vi "UHR-Fleezers Control (host) - Avogadro v2.vi"() -> ()   [LabVIEW 2014] (continued)
                                n2721 = local read "Confocal Y 1 (V)"() -> (w4187:dbl)
                                n2722 = property on="AO2" class="Slide (strict)"("Val(Sgnl)"=w4186) -> ()  [unwired: 2 in, 2 out]
                                n2723 = property on="AO1" class="Slide (strict)"("Val(Sgnl)"=w4187) -> ()  [unwired: 2 in, 2 out]
                                }
                                }
                                }
                                }
                                }
                                }
                                }
                                }
                                }
                                frame "Image" {
                                n2724 = property on="Confocal Image" class="Bool (strict)"("Val(Sgnl)"=TRUE ("Value (Signaling)")) -> ()  [unwired: 2 in, 2 out]
                                }
                              }
                              n2725 = local write "Fl. High"(FALSE ("Fl. High")) -> ()
                              n2726 = local read "Time (s)"() -> (w4123:dbl)
                            }
                            frame #1 {
                              n2727 = case shown="True" "Auto F Reset" {
                                tunnel: w4195 -> [_ w4200]
                                tunnel: w4194 -> [_ w4199]
                                tunnel: w4193 -> [_ w4198]
                                tunnel: w4192 -> [_ w4197]
                                frame False {
                                }
                                frame True {
                                n2728 = node-c288() -> (w4202:T42)  [unwired: 4 in]
                                n2729 = timed-loop {
                                timing: w4202 -> [_]
                                timing-out: [_] -> w4201
                                tunnel: w4200 -> [w4207]
                                tunnel: w4199 -> [w4206]
                                tunnel: w4198 -> [w4205]
                                tunnel: w4197 -> [w4204]
                                stop <- w4203 stop-if-true
                                n2730 = node-c288() -> ()  [unwired: 1 in, 1 out]
                                n2731 = local read "Fl. Delta Thresh. (kHz)"() -> (w4216:dbl)
                                n2732 = local read "APD to Watch"() -> (w4217:bool)
                                n2733 = local read "Delta Fl. 1"() -> (w4218:dbl)
                                n2734 = local read "Delta Fl. 2"() -> (w4219:dbl)
                                n2735 = local read "Fl. Triggered..."() -> (w4210:bool)
                                n2736 = local read "Stop All"() -> (w4211:bool)
                                n2737 = local read "Reset Force"() -> (w4209:bool)
                                n2738 = Multiply(x=w4216, y=1000.0) -> (x*y=w4214:dbl)
                                n2739 = Select(t=w4218, s=w4217, f=w4219) -> (s? t:f=w4213:dbl)
                                n2740 = Not(x=w4210) -> (.not. x?=w4208:bool)
                                n2741 = Greater?(x=w4213, y=w4214) -> (0:w4212:bool)
                                n2742 = Compound Arithmetic op=OR(w4212, w4211, w4208, w4209) -> (w4203:bool)
                                n2743 = case shown="True" w4203 {
                                tunnel: w4207 -> [_ w4223]
                                tunnel: w4206 -> [_ w4227]
                                tunnel: w4205 -> [_ w4226]
                                tunnel: w4204 -> [_ w4225]
                                frame False {
                                }
                                frame True {
                                n2744 = case shown="\"Yank\"" w4227 {
                                tunnel: w4226 -> [_ w4237]
                                tunnel: w4225 -> [_ w4235]
                                frame "Image", Default {
                                }
                                frame "Yank" {
                                n2745 = flat-sequence {
                                tunnel: [w4240] -> w4238
                                tunnel: w4237 -> [w4240]
                                tunnel: [w4239] -> w4236
                                tunnel: w4235 -> [w4239]
                                tunnel: w4238 -> [w4246]
                                tunnel: w4236 -> [w4244]
                                frame #0 {
                                n2746 = local read "Yank Delay (s)"() -> (w4243:dbl)
                                n2747 = Multiply(x=w4243, y=1000.0) -> (x*y=w4241:dbl)
                                n2748 = Wait (ms)(milliseconds to wait=w4241) -> ()  [unwired: 1 out]
                                }
                                frame #1 {
                                n2749 = local read "Yank to which?"() -> (w4245:bool)
                                n2750 = case shown="False" w4245 {
                                tunnel: w4246 -> [_ w4274]
                                tunnel: w4244 -> [w4247 _]
                                frame False {
                                n2751 = flat-sequence {
                                tunnel: w4247 -> [w4248]
                                frame #0 {
                                n2752 = property on="Trap Pos FB SP" class="DigNum (strict)"("Val(Sgnl)"=w4248) -> ()  [unwired: 2 in, 2 out]
                                }
                                frame #1 {
                                n2753 = Wait (ms)(milliseconds to wait=u32 700) -> ()  [unwired: 1 out]
                                }
                                frame #2 {
                                n2754 = local read "Action (%)"() -> (w4253:dbl)
                                n2755 = Absolute Value(x=w4253) -> (abs(x)=w4252:dbl)
                                n2756 = Greater?(x=w4252, y=70.0) -> (0:w4250:bool)
                                n2757 = property on="Remove Action Offset" class="Bool (strict)"("Val(Sgnl)"=w4250) -> ()  [unwired: 2 in, 2 out]
                                }
                                frame #3 {
                                n2758 = for {
                                N: 4 -> [_]
                                n2759 = flat-sequence {
                                frame #0 {
                                n2760 = Wait (ms)(milliseconds to wait=u32 500) -> ()  [unwired: 1 out]
                                }
                                frame #1 {
                                n2761 = local read "Action (%)"() -> (w4259:dbl)
                                n2762 = Absolute Value(x=w4259) -> (abs(x)=w4258:dbl)
                                n2763 = Greater?(x=w4258, y=70.0) -> (0:w4256:bool)
                                n2764 = property on="Remove Action Offset" class="Bool (strict)"("Val(Sgnl)"=w4256) -> ()  [unwired: 2 in, 2 out]
                                }
                                }
                                }
                                }
                                frame #4 {
                                n2765 = Wait (ms)(milliseconds to wait=u32 500) -> ()  [unwired: 1 out]
                                }
                                frame #5 {
                                n2766 = local read "Shift confocal"() -> (w4264:bool)
                                n2767 = local read "Mean"() -> (w4267:dbl)
                                n2768 = Greater?(x=w4267, y=11.0) -> (0:w4263:bool)
                                n2769 = Not(x=w4263) -> (.not. x?=w4262:bool)
                                n2770 = And(x=w4263, y=w4264) -> (x .and. y?=w4265:bool)
                                n2771 = And(x=w4262, y=w4264) -> (x .and. y?=w4261:bool)
                                n2772 = case shown="True" w4265 {
                                frame False {
                                }
                                frame True {
                                n2773 = local read "Confocal X 2 (V)"() -> (w4270:dbl)
                                n2774 = local read "Confocal Y 2 (V)"() -> (w4271:dbl)
                                n2775 = property on="AO2" class="Slide (strict)"("Val(Sgnl)"=w4270) -> ()  [unwired: 2 in, 2 out]
                                n2776 = property on="AO1" class="Slide (strict)"("Val(Sgnl)"=w4271) -> ()  [unwired: 2 in, 2 out]
                                }
                                }
                                n2777 = case shown="True" w4261 {
                                frame False {
                                }
                                frame True {
                                n2778 = local read "Confocal Y 1 (V)"() -> (w4269:dbl)
                                n2779 = local read "Confocal X 1 (V)"() -> (w4268:dbl)
                                n2780 = property on="AO1" class="Slide (strict)"("Val(Sgnl)"=w4269) -> ()  [unwired: 2 in, 2 out]
                                n2781 = property on="AO2" class="Slide (strict)"("Val(Sgnl)"=w4268) -> ()  [unwired: 2 in, 2 out]
                                }
                                }
                                }
                                frame #6 {
                                n2782 = Wait (ms)(milliseconds to wait=u32 1500) -> ()  [unwired: 1 out]
                                }
                                frame #7 {
                                n2783 = property on="Rem fb disp offset" class="Bool (strict)"("Val(Sgnl)"=TRUE ("Value (Signaling)")) -> ()  [unwired: 2 in, 2 out]
                                }
                                }
                                }
                                frame True {
                                n2784 = flat-sequence {
                                tunnel: w4274 -> [w4275]
                                frame #0 {
                                n2785 = property on="Trap Delta (MHz)" class="DigNum (strict)"("Val(Sgnl)"=w4275) -> ()  [unwired: 2 in, 2 out]
                                }
                                frame #1 {
                                n2786 = Wait (ms)(milliseconds to wait=u32 500) -> ()  [unwired: 1 out]
                                }
                                frame #2 {
                                n2787 = local read "Shift confocal"() -> (w4281:bool)
                                n2788 = local read "Mean"() -> (w4282:dbl)
                                n2789 = Greater?(x=w4282, y=11.0) -> (0:w4280:bool)
                                n2790 = And(x=w4280, y=w4281) -> (x .and. y?=w4278:bool)
                                n2791 = Not(x=w4280) -> (.not. x?=w4279:bool)
                                n2792 = And(x=w4279, y=w4281) -> (x .and. y?=w4277:bool)
                                n2793 = case shown="True" w4278 {
                                frame False {
                                }
                                frame True {
                                n2794 = local read "Confocal Y 2 (V)"() -> (w4287:dbl)
                                n2795 = local read "Confocal X 2 (V)"() -> (w4286:dbl)
                                n2796 = property on="AO1" class="Slide (strict)"("Val(Sgnl)"=w4287) -> ()  [unwired: 2 in, 2 out]
                                n2797 = property on="AO2" class="Slide (strict)"("Val(Sgnl)"=w4286) -> ()  [unwired: 2 in, 2 out]
                                }
                                }
                                n2798 = case shown="True" w4277 {
                                frame False {
                                }
                                frame True {
                                n2799 = local read "Confocal Y 1 (V)"() -> (w4285:dbl)
                                n2800 = local read "Confocal X 1 (V)"() -> (w4284:dbl)
                                n2801 = property on="AO2" class="Slide (strict)"("Val(Sgnl)"=w4284) -> ()  [unwired: 2 in, 2 out]
                                n2802 = property on="AO1" class="Slide (strict)"("Val(Sgnl)"=w4285) -> ()  [unwired: 2 in, 2 out]
                                }
                                }
                                }
                                }
                                }
                                }
                                }
                                }
                                }
                                }
                                n2803 = local read "Time (s)"() -> (w4222:dbl)
                                n2804 = Subtract(x=w4223, y=w4222) -> (x-y=w4234:dbl)
                                n2805 = Number To Decimal String(number=w4234, width (-)=i16 0) -> (decimal integer string=w4232:string)
                                n2806 = Concatenate Strings(w4232, " s fluorescence event") -> (w4229:string)
                                n2807 = local read "Messages"() -> (w4230:string)
                                n2808 = local write "Duration (s)"(w4234) -> ()
                                n2809 = call "Update messages.vi"("Message to add"=w4229, "Old message string"=w4230) -> ("New message string"=w4228:string)
                                n2810 = local write "Messages"(w4228) -> ()
                                n2811 = call <vilib>:"Beep.vi"() -> ()  [unwired: 12 in]
                                n2812 = local write "Reset Force"(FALSE ("Force Reset")) -> ()
                                n2813 = local write "Fl. High"(TRUE ("Fl. High")) -> ()
                                n2814 = local write "Waiting"(TRUE ("Waiting")) -> ()
                                }
                                }
                                n2815 = node-c288() -> ()  [unwired: 1 in, 1 out]
                                }
                                n2816 = node-c288(w4201) -> ()  [unwired: 1 out]
                                }
                              }
                            }
                          }
                          n2817 = local read "Trap Delta (MHz)"() -> (w4113:dbl)
                          n2818 = local read "Trap Pos FB SP"() -> (w4111:fxp<+/-,16,1>)
                        }
                      }
                    }
                    frame True {
                      n2819 = flat-sequence {
                        tunnel: w4298 -> [w4308]
                        tunnel: [w4308] -> w4302
                        tunnel: w4301 -> [w4307]
                        tunnel: [w4307] -> w4300
                        tunnel: [w4306] -> w4299
                        tunnel: w4297 -> [w4305]
                        tunnel: [w4304] -> w4296
                        tunnel: w4293 -> [w4303]
                        tunnel: [w4303] -> w4292
                        tunnel: w4302 -> [w4378]
                        tunnel: w4300 -> [w4377]
                        tunnel: w4299 -> [w4376]
                        tunnel: w4296 -> [w4375]
                        tunnel: w4292 -> [w4374]
                        tunnel: [w4375] -> w4295
                        frame #0 {
                          n2820 = call <vilib>:"Beep.vi"() -> ()  [unwired: 3 in, 9 out]
                          n2821 = local write "Waiting"(FALSE ("Waiting")) -> ()
                          n2822 = Increment(x=w4305) -> (x+1=w4304:u8)
                          n2823 = case shown="\"Image\"" w4307 {
                            tunnel: w4304 -> [_ _ w4314]
                            frame "Image" {
                              n2824 = property on="Confocal Image" class="Bool (strict)"("Val(Sgnl)"=TRUE ("Value (Signaling)")) -> ()  [unwired: 2 in, 2 out]
                            }
                            frame "Alarm", Default {
                            }
                            frame "Yank" {
                              n2825 = flat-sequence {
                                tunnel: w4314 -> [w4317]
                                tunnel: [w4316] -> w4313
                                tunnel: ["N Array El"] -> w4312
                                tunnel: w4313 -> [w4331]
                                tunnel: w4312 -> [w4327]
                                frame #0 {
                                n2826 = Multiply(x="Yank Delay (s)", y=1000.0) -> (x*y=w4320:dbl)
                                n2827 = Quotient & Remainder(x=w4317, y="N Array El") -> (x-y*floor(x/y)=w4316:u8)  [unwired: 1 out]
                                n2828 = Wait (ms)(milliseconds to wait=w4320) -> ()  [unwired: 1 out]
                                }
                                frame #1 {
                                n2829 = Random Number (0-1)() -> (number: 0 to 1=w4328:dbl)
                                n2830 = Multiply(x=w4327, y=w4328) -> (x*y=w4326:dbl)
                                n2831 = Round Toward -Infinity(1:w4326) -> (0:w4325:dbl)
                                n2832 = Select(t=w4325, s="Random Choice", f=w4331) -> (s? t:f=w4329:dbl)
                                n2833 = Select(t="Yank to Trap Delta (MHz)", s="Yank to which?", f="Yank to SP") -> (s? t:f=w4322:dbl[])
                                n2834 = Index Array(array=w4322, index=w4329) -> (element=w4332:dbl)
                                n2835 = case shown="False" "Yank to which?" {
                                tunnel: w4332 -> [w4333 w4359]
                                frame False {
                                n2836 = flat-sequence {
                                tunnel: w4333 -> [w4334]
                                frame #0 {
                                n2837 = property on="Trap Pos FB SP" class="DigNum (strict)"("Val(Sgnl)"=w4334) -> ()  [unwired: 2 in, 2 out]
                                }
                                frame #1 {
                                n2838 = Wait (ms)(milliseconds to wait=u32 700) -> ()  [unwired: 1 out]
                                }
                                frame #2 {
                                n2839 = local read "Action (%)"() -> (w4339:dbl)
                                n2840 = Absolute Value(x=w4339) -> (abs(x)=w4338:dbl)
                                n2841 = Greater?(x=w4338, y=70.0) -> (0:w4336:bool)
                                n2842 = property on="Remove Action Offset" class="Bool (strict)"("Val(Sgnl)"=w4336) -> ()  [unwired: 2 in, 2 out]
                                }
                                frame #3 {
                                n2843 = for {
                                N: 4 -> [_]
                                n2844 = flat-sequence {
                                frame #0 {
                                n2845 = Wait (ms)(milliseconds to wait=u32 500) -> ()  [unwired: 1 out]
                                }
                                frame #1 {
                                n2846 = local read "Action (%)"() -> (w4345:dbl)
                                n2847 = Absolute Value(x=w4345) -> (abs(x)=w4344:dbl)
                                n2848 = Greater?(x=w4344, y=70.0) -> (0:w4342:bool)
                                n2849 = property on="Remove Action Offset" class="Bool (strict)"("Val(Sgnl)"=w4342) -> ()  [unwired: 2 in, 2 out]
                                }
                                }
                                }
                                }
                                frame #4 {
                                n2850 = local read "Shift confocal"() -> (w4349:bool)
                                n2851 = local read "Mean"() -> (w4352:dbl)
                                n2852 = Greater?(x=w4352, y=11.0) -> (0:w4348:bool)
                                n2853 = Not(x=w4348) -> (.not. x?=w4347:bool)
                                n2854 = And(x=w4347, y=w4349) -> (x .and. y?=w4346:bool)
                                n2855 = And(x=w4348, y=w4349) -> (x .and. y?=w4350:bool)
                                n2856 = case shown="True" w4350 {
                                frame False {
                                }
                                frame True {
                                n2857 = local read "Confocal X 2 (V)"() -> (w4355:dbl)
                                n2858 = local read "Confocal Y 2 (V)"() -> (w4356:dbl)
                                n2859 = property on="AO2" class="Slide (strict)"("Val(Sgnl)"=w4355) -> ()  [unwired: 2 in, 2 out]
                                n2860 = property on="AO1" class="Slide (strict)"("Val(Sgnl)"=w4356) -> ()  [unwired: 2 in, 2 out]
                                }
                                }
                                n2861 = case shown="True" w4346 {
                                frame False {
                                }
                                frame True {
                                n2862 = local read "Confocal X 1 (V)"() -> (w4353:dbl)
                                n2863 = local read "Confocal Y 1 (V)"() -> (w4354:dbl)
                                n2864 = property on="AO1" class="Slide (strict)"("Val(Sgnl)"=w4354) -> ()  [unwired: 2 in, 2 out]
                                n2865 = property on="AO2" class="Slide (strict)"("Val(Sgnl)"=w4353) -> ()  [unwired: 2 in, 2 out]
                                }
                                }
                                }
                                frame #5 {
                                n2866 = Wait (ms)(milliseconds to wait=u32 1500) -> ()  [unwired: 1 out]
                                }
                                frame #6 {
                                n2867 = property on="Rem fb disp offset" class="Bool (strict)"("Val(Sgnl)"=TRUE ("Value (Signaling)")) -> ()  [unwired: 2 in, 2 out]
                                }
                                }
                                }
                                frame True {
                                n2868 = flat-sequence {
                                tunnel: w4359 -> [w4360]
                                frame #0 {
                                n2869 = property on="Trap Delta (MHz)" class="DigNum (strict)"("Val(Sgnl)"=w4360) -> ()  [unwired: 2 in, 2 out]
                                }
                                frame #1 {
                                n2870 = Wait (ms)(milliseconds to wait=u32 500) -> ()  [unwired: 1 out]
                                }
                                frame #2 {
                                n2871 = local read "Shift confocal"() -> (w4364:bool)
                                n2872 = local read "Mean"() -> (w4362:dbl)
                                n2873 = Greater?(x=w4362, y=11.0) -> (0:w4365:bool)
                                n2874 = Not(x=w4365) -> (.not. x?=w4366:bool)
                                n2875 = And(x=w4366, y=w4364) -> (x .and. y?=w4368:bool)
                                n2876 = And(x=w4365, y=w4364) -> (x .and. y?=w4367:bool)
                                n2877 = case shown="True" w4367 {
                                frame False {
                                }
                                frame True {
                                n2878 = local read "Confocal Y 2 (V)"() -> (w4372:dbl)
                                n2879 = local read "Confocal X 2 (V)"() -> (w4371:dbl)
                                n2880 = property on="AO1" class="Slide (strict)"("Val(Sgnl)"=w4372) -> ()  [unwired: 2 in, 2 out]
                                n2881 = property on="AO2" class="Slide (strict)"("Val(Sgnl)"=w4371) -> ()  [unwired: 2 in, 2 out]
                                }
                                }
                                n2882 = case shown="True" w4368 {
                                frame False {
                                }
                                frame True {
                                n2883 = local read "Confocal X 1 (V)"() -> (w4369:dbl)
                                n2884 = local read "Confocal Y 1 (V)"() -> (w4370:dbl)
                                n2885 = property on="AO2" class="Slide (strict)"("Val(Sgnl)"=w4369) -> ()  [unwired: 2 in, 2 out]
                                n2886 = property on="AO1" class="Slide (strict)"("Val(Sgnl)"=w4370) -> ()  [unwired: 2 in, 2 out]
                                }
                                }
                                }
                                }
                                }
                                }
                                }
                              }
                            }
                          }
                          n2887 = local read "Time (s)"() -> (w4306:dbl)
                          "Fl. High" <- TRUE ("Yanking")
                        }
                        frame #1 {
                          n2888 = local read "Auto F Reset"() -> (w4373:bool)
                          n2889 = case shown="True" w4373 {
                            tunnel: w4378 -> [_ w4382]
                            tunnel: w4377 -> [_ w4381]
                            tunnel: w4376 -> [_ w4380]
                            tunnel: w4374 -> [_ w4379]
                            frame False {
                            }
                            frame True {
                              n2890 = node-c288() -> (w4384:T42)  [unwired: 4 out]
                              n2891 = timed-loop {
                                timing: w4384 -> [_]
                                timing-out: [_] -> w4383
                                tunnel: w4382 -> [w4402]
                                tunnel: w4381 -> [w4401]
                                tunnel: w4380 -> [w4400]
                                tunnel: w4379 -> [w4399]
                                stop <- w4385 stop-if-true
                                n2892 = node-c288() -> ()  [unwired: 2 out]
                                n2893 = local read "Fl. Delta Thresh. (kHz)"() -> (w4393:dbl)
                                n2894 = local read "Fl. Triggered..."() -> (w4398:bool)
                                n2895 = local read "Delta Fl. 1"() -> (w4389:dbl)
                                n2896 = local read "Delta Fl. 2"() -> (w4387:dbl)
                                n2897 = local read "Stop All"() -> (w4396:bool)
                                n2898 = local read "APD to Watch"() -> (w4388:bool)
                                n2899 = Select(t=w4389, s=w4388, f=w4387) -> (s? t:f=w4386:dbl)
                                n2900 = Not(x=w4398) -> (.not. x?=w4397:bool)
                                n2901 = Multiply(x=w4393, y=1000.0) -> (x*y=w4392:dbl)
                                n2902 = Negate(x=w4392) -> (-x=w4391:dbl)
                                n2903 = Less?(x=w4386, y=w4391) -> (x < y?=w4395:bool)
                                n2904 = Compound Arithmetic op=OR(w4395, w4396, w4397, "Reset Force") -> (w4385:bool)
                                n2905 = case shown="True" w4385 {
                                tunnel: w4402 -> [_ w4417]
                                tunnel: w4401 -> [_ w4416]
                                tunnel: w4400 -> [_ w4406]
                                tunnel: w4399 -> [_ w4408]
                                frame False {
                                }
                                frame True {
                                n2906 = local read "Time (s)"() -> (w4407:dbl)
                                n2907 = case shown="\"Yank\"" w4416 {
                                tunnel: w4417 -> [_ w4420]
                                tunnel: w4408 -> [_ w4418]
                                frame "Image", Default {
                                }
                                frame "Yank" {
                                n2908 = flat-sequence {
                                tunnel: [w4426] -> w4421
                                tunnel: w4420 -> [w4426]
                                tunnel: [w4422] -> w4419
                                tunnel: w4418 -> [w4422]
                                tunnel: w4421 -> [w4429]
                                tunnel: w4419 -> [w4427]
                                frame #0 {
                                n2909 = local read "Yank Delay (s)"() -> (w4425:dbl)
                                n2910 = Multiply(x=w4425, y=1000.0) -> (x*y=w4423:dbl)
                                n2911 = Wait (ms)(milliseconds to wait=w4423) -> ()  [unwired: 1 out]
                                }
                                frame #1 {
                                n2912 = local read "Yank to which?"() -> (w4428:bool)
                                n2913 = case shown="False" w4428 {
                                tunnel: w4429 -> [_ w4456]
                                tunnel: w4427 -> [w4430 _]
                                frame False {
                                n2914 = flat-sequence {
                                tunnel: w4430 -> [w4431]
                                frame #0 {
                                n2915 = property on="Trap Pos FB SP" class="DigNum (strict)"("Val(Sgnl)"=w4431) -> ()  [unwired: 2 in, 2 out]
                                }
                                frame #1 {
                                n2916 = Wait (ms)(milliseconds to wait=u32 700) -> ()  [unwired: 1 out]
                                }
                                frame #2 {
                                n2917 = local read "Action (%)"() -> (w4436:dbl)
                                n2918 = Absolute Value(x=w4436) -> (abs(x)=w4435:dbl)
                                n2919 = Greater?(x=w4435, y=70.0) -> (0:w4433:bool)
                                n2920 = property on="Remove Action Offset" class="Bool (strict)"("Val(Sgnl)"=w4433) -> ()  [unwired: 2 in, 2 out]
                                }
                                frame #3 {
                                n2921 = for {
                                N: 4 -> [_]
                                n2922 = flat-sequence {
                                frame #0 {
                                n2923 = Wait (ms)(milliseconds to wait=u32 500) -> ()  [unwired: 1 out]
                                }
                                frame #1 {
                                n2924 = local read "Action (%)"() -> (w4442:dbl)
                                n2925 = Absolute Value(x=w4442) -> (abs(x)=w4441:dbl)
                                n2926 = Greater?(x=w4441, y=70.0) -> (0:w4439:bool)
                                n2927 = property on="Remove Action Offset" class="Bool (strict)"("Val(Sgnl)"=w4439) -> ()  [unwired: 2 in, 2 out]
                                }
                                }
                                }
                                }
                                frame #4 {
                                n2928 = local read "Shift confocal"() -> (w4447:bool)
                                n2929 = local read "Mean"() -> (w4449:dbl)
                                n2930 = Greater?(x=w4449, y=11.0) -> (0:w4446:bool)
                                n2931 = Not(x=w4446) -> (.not. x?=w4445:bool)
                                n2932 = And(x=w4446, y=w4447) -> (x .and. y?=w4444:bool)
                                n2933 = And(x=w4445, y=w4447) -> (x .and. y?=w4443:bool)
                                n2934 = case shown="True" w4444 {
                                frame False {
                                }
                                frame True {
                                n2935 = local read "Confocal Y 2 (V)"() -> (w4453:dbl)
                                n2936 = local read "Confocal X 2 (V)"() -> (w4452:dbl)
                                n2937 = property on="AO2" class="Slide (strict)"("Val(Sgnl)"=w4452) -> ()  [unwired: 2 in, 2 out]
                                n2938 = property on="AO1" class="Slide (strict)"("Val(Sgnl)"=w4453) -> ()  [unwired: 2 in, 2 out]
                                }
                                }
                                n2939 = case shown="True" w4443 {
                                frame False {
                                }
                                frame True {
                                n2940 = local read "Confocal X 1 (V)"() -> (w4450:dbl)
                                n2941 = local read "Confocal Y 1 (V)"() -> (w4451:dbl)
                                n2942 = property on="AO1" class="Slide (strict)"("Val(Sgnl)"=w4451) -> ()  [unwired: 2 in, 2 out]
                                n2943 = property on="AO2" class="Slide (strict)"("Val(Sgnl)"=w4450) -> ()  [unwired: 2 in, 2 out]
                                }
                                }
                                }
                                frame #5 {
                                n2944 = Wait (ms)(milliseconds to wait=u32 1500) -> ()  [unwired: 1 out]
                                }
                                frame #6 {
                                n2945 = property on="Rem fb disp offset" class="Bool (strict)"("Val(Sgnl)"=TRUE ("Value (Signaling)")) -> ()  [unwired: 2 in, 2 out]
                                }
                                }
                                }
                                frame True {
                                n2946 = flat-sequence {
                                tunnel: w4456 -> [w4457]
                                frame #0 {
                                n2947 = property on="Trap Delta (MHz)" class="DigNum (strict)"("Val(Sgnl)"=w4457) -> ()  [unwired: 2 in, 2 out]
                                }
                                frame #1 {
                                n2948 = Wait (ms)(milliseconds to wait=u32 500) -> ()  [unwired: 1 out]
                                }
                                frame #2 {
                                n2949 = local read "Shift confocal"() -> (w4463:bool)
                                n2950 = local read "Mean"() -> (w4465:dbl)
                                n2951 = Greater?(x=w4465, y=11.0) -> (0:w4462:bool)
                                n2952 = Not(x=w4462) -> (.not. x?=w4461:bool)
                                n2953 = And(x=w4462, y=w4463) -> (x .and. y?=w4460:bool)
                                n2954 = And(x=w4461, y=w4463) -> (x .and. y?=w4459:bool)
                                n2955 = case shown="True" w4460 {
                                frame False {
                                }
                                frame True {
                                n2956 = local read "Confocal Y 2 (V)"() -> (w4469:dbl)
                                n2957 = local read "Confocal X 2 (V)"() -> (w4468:dbl)
                                n2958 = property on="AO2" class="Slide (strict)"("Val(Sgnl)"=w4468) -> ()  [unwired: 2 in, 2 out]
                                n2959 = property on="AO1" class="Slide (strict)"("Val(Sgnl)"=w4469) -> ()  [unwired: 2 in, 2 out]
                                }
                                }
                                n2960 = case shown="True" w4459 {
                                frame False {
                                }
                                frame True {
                                n2961 = local read "Confocal Y 1 (V)"() -> (w4467:dbl)
                                n2962 = local read "Confocal X 1 (V)"() -> (w4466:dbl)
                                n2963 = property on="AO2" class="Slide (strict)"("Val(Sgnl)"=w4466) -> ()  [unwired: 2 in, 2 out]
                                n2964 = property on="AO1" class="Slide (strict)"("Val(Sgnl)"=w4467) -> ()  [unwired: 2 in, 2 out]
                                }
                                }
                                }
                                }
                                }
                                }
                                }
                                }
                                }
                                }
                                n2965 = local read "Messages"() -> (w4415:string)
                                n2966 = Subtract(x=w4407, y=w4406) -> (x-y=w4413:dbl)
                                "Duration (s)" <- w4413
                                n2967 = Number To Decimal String(number=w4413, width (-)=i16 0) -> (decimal integer string=w4411:string)
                                n2968 = Concatenate Strings(w4411, " s fluorescence event." ("string")) -> (w4409:string)
                                n2969 = call "Update messages.vi"("Message to add"=w4409, "Old message string"=w4415) -> ("New message string"=w4414:string)
                                n2970 = local write "Reset Force"(FALSE ("Reset Force")) -> ()
                                n2971 = local write "Waiting"(TRUE ("Waiting")) -> ()
                                n2972 = local write "Messages"(w4414) -> ()
                                n2973 = local write "Fl. High"(FALSE ("Fl. High")) -> ()
                                n2974 = call <vilib>:"Beep.vi"() -> ()  [unwired: 3 in, 9 out]
                                }
                                }
                                n2975 = node-c288() -> ()  [unwired: 2 out]
                              }
                              n2976 = node-c288(w4383) -> ()  [unwired: 1 out]
                            }
                          }
                        }
                      }
                      n2977 = local read "Trap Delta (MHz)"() -> (w4298:dbl)
                      n2978 = local read "Trap Pos FB SP"() -> (w4293:fxp<+/-,16,1>)
                    }
                  }
                }
                frame #1 {
                  n2979 = local read "Stop All"() -> (w4479:bool)
                  n2980 = local read "Fl. Triggered..."() -> (w4477:bool)
                  n2981 = Not(x=w4477) -> (.not. x?=w4478:bool)
                  n2982 = Or(x=w4478, y=w4479) -> (x .or. y?=w4476:bool)
                }
              }
              n2983 = case shown="True" w4070 {
                frame False {
                }
                frame True {
                  n2984 = local read "Confocal Y 1 (V)"() -> (w4080:dbl)
                  n2985 = local read "Confocal X 1 (V)"() -> (w4079:dbl)
                  n2986 = property on="AO2" class="Slide (strict)"("Val(Sgnl)"=w4079) -> ()  [unwired: 2 in, 2 out]
                  n2987 = property on="AO1" class="Slide (strict)"("Val(Sgnl)"=w4080) -> ()  [unwired: 2 in, 2 out]
                }
              }
              n2988 = case shown="True" w4070 {
                frame False {
                }
                frame True {
                  w4078 = FALSE ("Fl. High")
                  n2989 = local write "Waiting"(w4078) -> ()
                  n2990 = local write "Fl. High"(w4078) -> ()
                }
              }
              n2991 = node-c288() -> ()  [unwired: 2 out]
            }
            n2992 = node-c288(w4068) -> ()  [unwired: 1 out]
          }
        }
      }
      event "Start assembly line": Value Change {
        n2993 = event-data() -> ()  [unwired: 7 out]
        n2994 = case shown="True" "Start assembly line" {
          tunnel: w4485 -> [_ w4486]
          frame False {
          }
          frame True {
            n2995 = flat-sequence {
              tunnel: w4486 -> [w4491]
              tunnel: [w4490] -> w4488
              tunnel: w4488 -> [w4523]
              tunnel: [w4522] -> w4487
              tunnel: w4487 -> [w4525]
              tunnel: w4486 -> [w4544]
              frame #0 {
                w4489 = TRUE ("Value (Signaling)")
                n2996 = property on="Green Laser ON" class="Bool (strict)"("Val(Sgnl)"=w4489) -> ()  [unwired: 2 in, 2 out]
                "AL Running" <- w4489
              }
              frame #1 {
                n2997 = node-c288() -> (w4493:T42)  [unwired: 4 in]
                n2998 = timed-loop {
                  timing: w4493 -> [_]
                  timing-out: [_] -> w4492
                  tunnel: w4491 -> [w4501]
                  tunnel: [w4496] -> w4490
                  stop <- w4497 stop-if-true
                  n2999 = node-c288() -> ()  [unwired: 1 in, 1 out]
                  n3000 = local read "APD rates cluster"() -> (w4495:T2)
                  n3001 = Multiply(x="Cy3 Fl.  Thresh. (kHz)", y=1000.0) -> (x*y=w4504:dbl)
                  n3002 = Unbundle By Name(w4495) -> ("APD 1 Rate (Hz)"=w4494:dbl)
                  n3003 = Greater?(x=w4494, y=w4504) -> (0:w4500:bool)
                  n3004 = case shown="True" w4500 {
                    tunnel: w4501 -> [_ w4507]
                    tunnel: [TRUE ("Stage Moving") w4506] -> w4499
                    frame False {
                    }
                    frame True {
                      n3005 = flat-sequence {
                        tunnel: w4507 -> [w4512]
                        tunnel: [w4517] -> w4506
                        frame #0 {
                          n3006 = Multiply(x="AL Delay (s)", y=u32 1000) -> (x*y=w4509:u32)
                          n3007 = Wait (ms)(milliseconds to wait=w4509) -> ()  [unwired: 1 out]
                        }
                        frame #1 {
                          n3008 = property on="Green Laser ON" class="Bool (strict)"("Val(Sgnl)"=FALSE ("Value (Signaling)")) -> ()  [unwired: 2 in, 2 out]
                        }
                        frame #2 {
                          # "upper spot"
                          n3009 = local read "Saved Stage Positions"() -> (w4515:dbl[][])
                          n3010 = local write "Stage Moving"(TRUE ("Stage Moving")) -> ()
                          n3011 = call "move to saved stage position.vi"("Stage VISA resource name in"=w4512, "Position"=5, "Saved Stage Positions"=w4515) -> ("error out"=w4513:errorcluster)  [unwired: 1 in, 1 out]
                          n3012 = local write "Stage Control Serial Error"(w4513) -> ()
                        }
                        frame #3 {
                          w4517 = FALSE ("Stage Moving")
                          n3013 = call <vilib>:"Beep.vi"() -> ()  [unwired: 3 in, 9 out]
                          n3014 = local write "Stage Moving"(w4517) -> ()
                        }
                      }
                    }
                  }
                  n3015 = local read "Stop assembly line"() -> (w4496:bool)
                  n3016 = Not(x=w4499) -> (.not. x?=w4498:bool)
                  n3017 = node-c288() -> ()  [unwired: 1 in, 1 out]
                  n3018 = Or(x=w4498, y=w4496) -> (x .or. y?=w4497:bool)
                }
                n3019 = node-c288(w4492) -> ()  [unwired: 1 out]
              }
              frame #2 {
                n3020 = Not(x=w4523) -> (.not. x?=w4522:bool)
                n3021 = case shown="True" w4522 {
                  frame False {
                  }
                  frame True {
                    n3022 = property on="Red Laser ON" class="Bool (strict)"("Val(Sgnl)"=TRUE ("Value (Signaling)")) -> ()  [unwired: 2 in, 2 out]
                  }
                }
              }
              frame #3 {
                n3023 = node-c288() -> (w4527:T42)  [unwired: 4 in]
                n3024 = timed-loop {
                  timing: w4527 -> [_]
                  timing-out: [_] -> w4526
                  tunnel: [w4530] -> _
                  tunnel: w4525 -> [w4530]
                  stop <- "Stop assembly line" stop-if-true
                  n3025 = node-c288() -> ()  [unwired: 1 in, 1 out]
                  n3026 = local read "APD rates cluster"() -> (w4529:T2)
                  n3027 = Multiply(x="Cy5 Fl.  Thresh. (kHz)", y=1000.0) -> (x*y=w4536:dbl)
                  n3028 = Unbundle By Name(w4529) -> ("APD 2 Rate (Hz)"=w4528:dbl)
                  n3029 = Greater?(x=w4528, y=w4536) -> (0:w4533:bool)
                  n3030 = And(x=w4533, y=w4530) -> (x .and. y?=w4531:bool)
                  n3031 = case shown="True" w4531 {
                    frame False {
                    }
                    frame True {
                      n3032 = property on="Green Laser ON" class="Bool (strict)"("Val(Sgnl)"=TRUE ("Value (Signaling)")) -> ()  [unwired: 2 in, 2 out]
                    }
                  }
                  n3033 = node-c288() -> ()  [unwired: 1 in, 1 out]
                }
                n3034 = node-c288(w4526) -> ()  [unwired: 1 out]
              }
              frame #4 {
                w4543 = FALSE ("Value (Signaling)")
                # "lower spot"
                n3035 = local read "Saved Stage Positions"() -> (w4547:dbl[][])
                n3036 = property on="Red Laser ON" class="Bool (strict)"("Val(Sgnl)"=w4543) -> ()  [unwired: 2 in, 2 out]
                n3037 = property on="Green Laser ON" class="Bool (strict)"("Val(Sgnl)"=w4543) -> ()  [unwired: 2 in, 2 out]
                n3038 = local write "Stage Moving"(TRUE ("Stage Moving")) -> ()
                n3039 = local write "Stop assembly line"(FALSE ("Stop assembly line")) -> ()
                n3040 = call "move to saved stage position.vi"("Stage VISA resource name in"=w4544, "Position"=3, "Saved Stage Positions"=w4547) -> ("error out"=w4546:errorcluster)  [unwired: 1 in, 1 out]
                n3041 = local write "Stage Control Serial Error"(w4546) -> ()
              }
              frame #5 {
                w4549 = FALSE ("Stage Moving")
                n3042 = local write "Stage Moving"(w4549) -> ()
                n3043 = local write "AL Running"(w4549) -> ()
                n3044 = call <vilib>:"Beep.vi"() -> ()  [unwired: 3 in, 9 out]
              }
            }
          }
        }
      }
      event "Stop All": Value Change {
        n3045 = event-data() -> ()  [unwired: 7 out]
        n3046 = local read "Stop All"() -> (w4550:bool)
      }
    }
    n3047 = node-c288() -> ()  [unwired: 2 out]
  }
  n3048 = node-c288(w52) -> ()  [unwired: 1 out]
  n3049 = node-c288(w63) -> ()  [unwired: 1 out]
  n3050 = node-c288(w61) -> ()  [unwired: 1 out]
  n3051 = property on="Saved trap pos" class="WFGraph (strict)"("Visible"=FALSE) -> ()  [unwired: 2 in, 2 out]
  n3052 = property on="Trap Delta Graph" class="WFGraph (strict)"("Visible"=TRUE) -> ()  [unwired: 2 in, 2 out]
  n3053 = disable-structure shown="Disabled" {
    disable-tunnel: w55 -> [w4552 _]
    disable-tunnel: w54 -> [w4551 _]
    frame Disabled {
      n3054 = VISA Close(VISA resource name=w4552, error in (no error)=w4551) -> (error out=w4553:errorcluster)
      n3055 = call <vilib>:"Simple Error Handler.vi"("error in (no error)"=w4553) -> ()  [unwired: 1 in, 8 out]
    }
    frame Enabled {
    }
  }
  n3056 = disable-structure shown="Disabled" {
    disable-tunnel: [w4561 _] -> w20
    disable-tunnel: [w4557 _] -> w19
    disable-tunnel: [w4556 _] -> w18
    disable-tunnel: [w4555 _] -> w17
    disable-tunnel: [w4554 _] -> w16
    frame Disabled {
      # "n samples needed for data"
      n3057 = Unbundle By Name("sound format") -> ("sample rate (S/s)"=w4557:dbl)
      n3058 = call <vilib>:"Sound Output Configure.vi"("number of samples/ch"="number of samples/ch", "sample mode"="sample mode", "sound format"="sound format", "device ID"="device ID") -> ("task ID"=w4561:T60)  [unwired: 6 in, 1 out]
      n3059 = local read "DMA Update Period (s)"() -> (w4558:dbl)
      n3060 = Multiply(x=w4558, y=w4557) -> (x*y=w4556:dbl)
      n3061 = for "Sound time base" {
        N: w4556 -> [_]
        tunnel: [w4565] -> w4559 mode=indexing
        i -> [w4565]
      }
      n3062 = Reciprocal(x=w4557) -> (1/x=w4555:dbl)
      n3063 = Multiply(x=w4559, y=w4555) -> (x*y=w4554:dbl[])
    }
    frame Enabled {
    }
  }
  n3064 = timed-loop "Main data acquisition loop (get data, process data for display, and save data to disk)" {
    tunnel: w15 -> [w4700]
    tunnel: w28 -> [w4699]
    tunnel: [w4887] -> w75
    tunnel: [w4882] -> w74
    timing: w68 -> [_]
    timing-out: [_] -> w67
    tunnel: w46 -> [w4815]
    tunnel: [w4729] -> w21
    tunnel: w20 -> [w4728]
    tunnel: w19 -> [w4726]
    tunnel: w18 -> [w4725]
    tunnel: w17 -> [w4724]
    tunnel: w16 -> [w4723]
    stop <- "Stop All" stop-if-true
    w4643 = 3276.7
    w4772 = "Initialize"
    # "Modified by Ronen 180227: Allows for taking confocal image by moving the piezo trap with a bead inside and using trap 1 (AOM) with very low intensity to measure it"
    # "Cursor control of MCL trap position"
    # "Values for plotting"
    # "List of channels in order (X or Y only):\nT1 X (mV)\nT2 X (mV)\nT1 X (nm)\nT2 X (nm)\nT1 FX (pN)\nT2 FX (pN)\nPosition Difference (nm)\nAPD1\nAPD2\nAPD3"
    # "T2 sum"
    # "T1 sum"
    n3065 = node-c288() -> ()  [unwired: 2 out]
    n3066 = First Call?() -> (First Call?: T/F=w4784:bool)
    n3067 = Or(x="Reset", y=w4784) -> (x .or. y?=w4785:bool)
    n3068 = Or(x="Start AOD Scan", y="Trap Raster Scan") -> (x .or. y?=w4843:bool)
    n3069 = case "Reset data stream (manual reset or at begining of some rastering and imaging)" shown="True" w4785 {
      tunnel: w4700 -> [w5756 w5764]
      tunnel: w4699 -> [w5755 w5763]
      tunnel: [w5756 w5758] -> w4719
      tunnel: [w5755 w5757] -> w4720
      frame False {
      }
      frame True {
        w5761 = TRUE ("AI to FIFO")
        n3070 = call "reset FPGA DMA.vi"("error in"=w5763, "FPGA VI Reference In"=w5764) -> ("error out"=w5759:errorcluster, "FPGA VI Reference Out"=w5760:T40)
        n3071 = local write "Overflow (data lost)"(FALSE ("Overflow (data lost)")) -> ()
        n3072 = xnode "Read/Write Control"("FPGA VI Reference In"=w5760, "error in"=w5759, "AI to FIFO"=w5761, "APD to FIFO"=w5761) -> ("FPGA VI Reference Out"=w5758:T40, "error out"=w5757:errorcluster)
      }
    }
    n3073 = case "Start active calibration (oscillate traps precisely)" shown="True" "Active Cal" {
      tunnel: w4720 -> [w5086 w5094]
      tunnel: w4719 -> [w5085 w5095]
      tunnel: [w5086 w5091] -> w4718
      tunnel: [w5085 w5092] -> w4717
      frame False {
      }
      frame True {
        w5087 = TRUE ("APD to FIFO")
        n3074 = call "reset FPGA DMA.vi"("error in"=w5094, "FPGA VI Reference In"=w5095) -> ("error out"=w5088:errorcluster, "FPGA VI Reference Out"=w5089:T40)
        n3075 = local write "Active Cal"(FALSE ("Active Cal")) -> ()
        n3076 = local write "Save Calibration"(TRUE ("Save Calibration")) -> ()
        n3077 = xnode "Read/Write Control"("FPGA VI Reference In"=w5089, "error in"=w5088, "AI to FIFO"=w5087, "APD to FIFO"=w5087) -> ("FPGA VI Reference Out"=w5092:T40, "error out"=w5091:errorcluster)
      }
    }
    n3078 = case shown="True" "Read Lateness and Rel Phase" {
      tunnel: w4700 -> [w5300 w5331]
      tunnel: w4699 -> [w5301 w5330]
      tunnel: [w5300 w5302] -> w4675
      tunnel: [w5301 w5303] -> w4837
      frame False {
      }
      frame True {
        n3079 = xnode "Read/Write Control"("FPGA VI Reference In"=w5331, "error in"=w5330) -> ("FPGA VI Reference Out"=w5302:T40, "error out"=w5303:errorcluster, "GI Relative phase"=→"GI relative phase":i16, "Relative phase"=→"Relative phase (AI1)":i16, "AI Late Counter"=→"Late Counter (AI1)":u8, "GI Late Counter"=→"GI Late Counter":u8, "MCL Late Counter"=→"MCL Late Counter":u8, "MCL Relative Phase"=→"Relative Phase (MCL)":i16, "APD Acq Relative Phase"=→"APD Acq Relative Phase":i16, "APD 1 Gate Relative Phase"=→"APD 1 Gate Relative Phase":i16, "APD 2 Gate Relative Phase"=→"APD 2 Gate Relative Phase":i16, "APD Acq Late Counter"=→"APD Acq Late Counter":u8, "APD 1 Gate Late Counter"=→"APD 1 Gate Late Counter":u8, "APD 2 Gate Late Counter"=→"APD 2 Gate Late Counter":u8, "Green FB Relative Phase"=→"Relative phase (Green FB)":i16, "GI Relative phase 2"=→"GI relative phase 2":i16, "GI Late Counter 2"=→"GI Late Counter 2":u8, "Trap Pos FIFO Timeout"=→"Trap Pos FIFO Timeout":u16, "Trap AI FIFO Timeout"=→"Trap AI FIFO Timeout":u16, "RI Late Counter"=→"RI Late Counter":u8, "RI Relative phase"=→"RI relative phase":i16, "Green Late Counter"=→"Green AI Late Counter":u8, "BI Late Counter (AO)"=→"Late Counter (BI AO)":u8, "Blue Late Counter (D)"=→"Late Counter (BI DO)":u8, "BI Relative phase (AO)"=→"Relative phase (BI AO)":i16, "BI Relative phase (D)"=→"Relative phase (BI DO)":i16, "APD 3 Gate Late Counter"=→"APD 3 Gate Late Counter":u8, "APD 3 Gate Relative Phase"=→"APD 3 Gate Relative Phase":i16)
      }
    }
    n3080 = Compound Arithmetic op=OR("Start MCL Scan", "Confocal Image", "Confocal Linescan") -> (w4698:bool)
    n3081 = And(x="Save Data (MCL)", y=w4698) -> (x .and. y?=w4860:bool)
    n3082 = case "Start AOM raster scan" shown="True" w4843 {
      tunnel: w4717 -> [w5615 w5625]
      tunnel: w4718 -> [w5614 w5624]
      tunnel: [w5615 w5618] -> w4863
      tunnel: [w5614 w5617] -> w4862
      frame False {
      }
      frame True {
        n3083 = case shown="True" "Restart DMA? (AOD)" {
          tunnel: [w5654 w5656] -> w5619
          tunnel: [w5653 w5655] -> w5620
          tunnel: w5625 -> [w5654 w5658]
          tunnel: w5624 -> [w5653 w5657]
          frame False {
          }
          frame True {
            n3084 = local write "Overflow (data lost)"(FALSE ("Overflow (data lost)")) -> ()
            n3085 = call "reset FPGA DMA.vi"("error in"=w5657, "FPGA VI Reference In"=w5658) -> ("error out"=w5655:errorcluster, "FPGA VI Reference Out"=w5656:T40)
          }
        }
        n3086 = local write "Trap Raster Scan"(FALSE ("Trap Raster Scan")) -> ()
        n3087 = case shown="False" "Move MCL Also?" {
          tunnel: w5620 -> [w5628 w5648]
          tunnel: w5619 -> [w5629 w5649]
          tunnel: [w5627 w5652] -> w5618
          tunnel: [w5626 w5651] -> w5617
          frame False {
            w5630 = TRUE ("AI to FIFO")
            n3088 = xnode "Read/Write Control"("FPGA VI Reference In"=w5629, "error in"=w5628, "AI to FIFO"=w5630, "APD to FIFO"=w5630, "Start scan"=w5630) -> ("FPGA VI Reference Out"=w5627:T40, "error out"=w5626:errorcluster)
          }
          frame True {
            w5646 = FALSE ("1D or 2D Scan?")
            w5650 = TRUE ("AI to FIFO")
            n3089 = local read "Scan Range (nm)"() -> (w5643:dbl)
            n3090 = local read "Scan steps (AOD)"() -> (w5637:u64)
            n3091 = local read "Total Counts (ticks)"() -> (w5638:u16)
            n3092 = local read "Cycles/step (AOD)"() -> (w5636:u64)
            n3093 = local read "Number of F/B Scans (AOD)"() -> (w5645:u16)
            n3094 = Bundle("Scan Range (nm)"=w5643, "MCL Step Position Ratio"="MCL Step Position Ratio", "MCL/AOM Scale Tweak"="MCL/AOM Scale Tweak", "MCL X Cal (nm/V)"="MCL X Cal (nm/V)", "MCL Step Increment (V_int)"="MCL Step Increment (V_int)", "Total Counts (ticks)"=w5638, "Scan steps (AOD)"=w5637, "Cycles/step (AOD)"=w5636) -> (w5635:T65)  [unwired: 1 in]
            n3095 = call "Calculate MCL scan parameters.vi"("Input parameters"=w5635) -> ("Scan steps(MCL)"=w5634:dbl, "Scan Freq. Increment (MCL)"=w5633:dbl, "MCL Count"=w5632:dbl)
            "MCL Count" <- w5632
            n3096 = xnode "Read/Write Control"("FPGA VI Reference In"=w5649, "error in"=w5648, "Scan steps (MCL)"=w5634, "Number of scans (MCL)"=w5645, "Cycles per step (MCL)"=u64 1, "Scan freq.  increment (MCL)"=w5633, "1D or 2D Scan?"=w5646, "MCL Scan Axis"=w5646, "Cont. Scan (MCL)"=w5646, "MCL count"=w5632) -> ("FPGA VI Reference Out"=w5631:T40, "error out"=w5647:errorcluster)
            n3097 = local write "MCL Scanning"(w5650) -> ()
            n3098 = local write "wait to reset values"(w5650) -> ()
            n3099 = xnode "Read/Write Control"("FPGA VI Reference In"=w5631, "error in"=w5647, "AI to FIFO"=w5650, "APD to FIFO"=w5650, "Start scan"=w5650, "Start scan (MCL)"=w5650) -> ("FPGA VI Reference Out"=w5652:T40, "error out"=w5651:errorcluster)
          }
        }
        "Raster Scanning..." <- TRUE ("Scanning...")
      }
    }
    n3100 = case "Start MCL raster scan" shown="True" w4698 {